vi "Core_Chem_User_Interface_v1.4.vi"() -> ()   [LabVIEW 2014] (continued)
    n188 = Decimal String To Number(string=w445) -> (number=w443:i32)  [unwired: 2 in, 1 out]
    n189 = call "Find_Data_SubVI.vi"("FGGA"=w553, "CO"=w552, "Ozone"=w551, "SO2"=w472) -> ("Output Value"=→"CPU Total %":dbl)  [unwired: 11 in]
    n190 = call "Find_Data_SubVI.vi"("FGGA"=w541, "CO"=w540, "Ozone"=w539, "SO2"=w538) -> ("Output Value"=→"MFM":dbl)  [unwired: 11 in]
    n191 = call "Find_Data_SubVI.vi"("FGGA"=w536, "CO"=w535, "Ozone"=w534, "SO2"=w533) -> ("Output Value"=w532:dbl)  [unwired: 11 in]
    n192 = call "Find_Data_SubVI.vi"("FGGA"=w521, "CO"=w524, "Ozone"=w519, "SO2"=w526) -> ("Output Value"=→"USB Disk Space Used %":dbl)  [unwired: 11 in]
    n193 = Not Equal To 0?(x=w532) -> (x != 0?=→"PTP Sync":bool)
    n194 = Add(x=w443, y=u32 2082844800) -> (x+y=w442:u32)
    n195 = Scan Value(string=w403, format string="%f") -> (value=→"MFC1 Cal Flow":dbl)  [unwired: 1 in, 1 out]
    n196 = Scan Value(string=w367, format string="%f") -> (value=w365:dbl)  [unwired: 1 in, 1 out]
    n197 = Scan Value(string=w366, format string="%f") -> (value=w363:dbl)  [unwired: 1 in, 1 out]
    n198 = Scan Value(string=w416, format string="%f") -> (value=→"Cell temperature":dbl)  [unwired: 1 in, 1 out]
    n199 = Scan Value(string=w417, format string="%f") -> (value=→"Cell pressure":dbl)  [unwired: 1 in, 1 out]
    n200 = Scan Value(string=w422, format string="%f") -> (value=→"CH4 Dry":dbl)  [unwired: 1 in, 1 out]
    n201 = Scan Value(string=w425, format string="%f") -> (value=→"CO2 Dry":dbl)  [unwired: 1 in, 1 out]
    n202 = Scan Value(string=w427, format string="%f") -> (value=→"H2O":dbl)  [unwired: 1 in, 1 out]
    n203 = Scan Value(string=w432, format string="%f") -> (value=→"CO2":dbl)  [unwired: 1 in, 1 out]
    n204 = Scan Value(string=w435, format string="%f") -> (value=→"CH4":dbl)  [unwired: 1 in, 1 out]
    n205 = Scan Value(string=w563, format string="%f") -> (value=→"Std\nContent (barG)":dbl)  [unwired: 1 in, 1 out]
    n206 = Scan Value(string=w523, format string="%d", default (0 dbl)=u32 0) -> (value=w577:u32)  [unwired: 1 out]
    n207 = Scan Value(string=w562, format string="%f") -> (value=→"N2\nContent (barG)":dbl)  [unwired: 1 in, 1 out]
    n208 = Scan Value(string=w564, format string="%f") -> (value=→"CO2\nContent (barG)":dbl)  [unwired: 1 in, 1 out]
    n209 = Scan Value(string=w570, format string="%f") -> (value=→"CO2 Pressure\nDelivery (PSIA)":dbl)  [unwired: 1 in, 1 out]
    n210 = To Time Stamp(1:w442) -> (0:w448:timestamp)
    n211 = Scan Value(string=w511, format string="%f") -> (value=→"Lamp Flow Controller":dbl)  [unwired: 1 in, 1 out]
    n212 = Scan Value(string=w380, format string="%f") -> (value=→"Raw Signal":dbl)  [unwired: 1 in, 1 out]
    n213 = Scan Value(string=w374, format string="%f") -> (value=→"Lamp Temperature":dbl)  [unwired: 1 in, 1 out]
    n214 = Scan Value(string=w399, format string="%f") -> (value=→"CO Concentration":dbl)  [unwired: 1 in, 1 out]
    n215 = Scan Value(string=w508, format string="%f") -> (value=→"Monochromator Flow":dbl)  [unwired: 1 in, 1 out]
    n216 = Scan Value(string=w507, format string="%f") -> (value=→"Fluorescence Cell Pressure":dbl)  [unwired: 1 in, 1 out]
    n217 = Not Equal To 0?(x=w577) -> (x != 0?=→"CO CAL Status":bool)
    n218 = call "ping.vi"("host"="192.168.101.17" ("Host IP Address")) -> ("found?"=w372:bool)  [unwired: 8 in, 2 out]
    n219 = Scan Value(string=w490, format string="%f") -> (value=→"TEI49C Sample Flow B":dbl)  [unwired: 1 in, 1 out]
    n220 = Scan Value(string=w492, format string="%f") -> (value=→"TEi49C Concentration":dbl)  [unwired: 1 in, 1 out]
    n221 = Scan Value(string=w491, format string="%f") -> (value=→"TEI49C Sample Flow A":dbl)  [unwired: 1 in, 1 out]
    n222 = Scan Value(string=w467, format string="%f") -> (value=w458:dbl)  [unwired: 1 in, 1 out]
    n223 = Scan Value(string=w466, format string="%f") -> (value=w451:dbl)  [unwired: 1 in, 1 out]
    n224 = Not Equal?(x=w457, y=w458) -> (x != y?=w463:bool)
    n225 = Not Equal?(x=w449, y=w451) -> (x != y?=w456:bool)
    n226 = case shown="True" w463 {
      tunnel: w464 -> [w638 w647]
      tunnel: w462 -> [w639 w646]
      tunnel: [w639 w645] -> w461
      tunnel: w448 -> [_ w641]
      tunnel: w458 -> [_ w642]
      tunnel: [w638 w644] -> w460
      tunnel: [w637 w643] -> w459
      tunnel: w458 -> [_ w643]
      tunnel: w457 -> [w637 _]
      frame False {
      }
      frame True {
        n227 = Bundle(w641, w642) -> (w640:cluster{timestamp, dbl})  [unwired: 1 in]
        n228 = Replace Array Subset(array=w647, new element=w640, index=w646) -> (w644:cluster{"time stamp":timestamp, "Y":dbl}[])
        n229 = Increment(x=w646) -> (x+1=w645:i32)
      }
    }
    "CO Sensitivity" <- w460
    n230 = case shown="True" w456 {
      tunnel: w455 -> [w627 w636]
      tunnel: w454 -> [w628 w635]
      tunnel: [w628 w634] -> w452
      tunnel: w448 -> [_ w633]
      tunnel: w451 -> [_ w632]
      tunnel: [w627 w631] -> w453
      tunnel: [w626 w630] -> w450
      tunnel: w451 -> [_ w630]
      tunnel: w449 -> [w626 _]
      frame False {
      }
      frame True {
        n231 = Bundle(w633, w632) -> (w629:cluster{timestamp, dbl})  [unwired: 1 in]
        n232 = Replace Array Subset(array=w636, new element=w629, index=w635) -> (w631:cluster{"time stamp":timestamp, "Y":dbl}[])
        n233 = Increment(x=w635) -> (x+1=w634:i32)
      }
    }
    "CO Zero" <- w453
    n234 = case shown="True" w372 {
      tunnel: w447 -> [_ w625]
      tunnel: [FALSE w622] -> w446
      frame False {
      }
      frame True {
        n235 = Select(t=FALSE, s=w625, f=TRUE) -> (s? t:f=w622:bool)
      }
    }
    "Network to cRIO live status" <- w446
    n236 = Bundle(w365, w363) -> (→"Ring Down Time RDA & RDB":cluster{dbl, dbl})  [unwired: 1 in]
    n237 = Wait (ms)(milliseconds to wait=u32 1000) -> ()  [unwired: 1 out]
  }
  n238 = while {
    stop <- FALSE stop-if-true
    # "Preflight Sub VI Descriptions"
    n239 = Wait (ms)(milliseconds to wait=u32 500) -> ()  [unwired: 1 out]
    n240 = case shown="True" "Line Lock Setting Change" {
      frame False {
      }
      frame True {
        n241 = call "FGGA Linelock Settings Procedures.vi"() -> ()  [unwired: 12 in]
      }
    }
  }
  n242 = while {
    stop <- FALSE stop-if-true
    # "Postflight Sub VI Descriptions"
    n243 = case shown="True" "Postflight Procedures" {
      frame False {
      }
      frame True {
        n244 = call "PostFlight Procedures.vi"() -> ()  [unwired: 12 in]
      }
    }
    n245 = Wait (ms)(milliseconds to wait=u32 500) -> ()  [unwired: 1 out]
  }
  n246 = while {
    stop <- FALSE stop-if-true
    # "Preflight Sub VI Descriptions"
    n247 = case shown="True" "Prepare Gases" {
      frame False {
      }
      frame True {
        n248 = call "CO Gas Preparation.vi"() -> ()  [unwired: 12 in]
      }
    }
    n249 = Wait (ms)(milliseconds to wait=u32 500) -> ()  [unwired: 1 out]
  }
  n250 = Obtain Queue(name (unnamed)="FGGA_Command", element data type=w55) -> (queue out=w2:refnum<queue>, error out=w1:errorcluster)  [unwired: 3 in, 1 out]
  n251 = while {
    shift-right: [w660] -> _
    shift-left: u8 1 -> [w661]
    tunnel: w2 -> [w658]
    tunnel: w1 -> [w657]
    stop <- FALSE stop-if-true
    # "FGGA pump synchronise to WoW Wait on Wheel Flag"
    n252 = Wait (ms)(milliseconds to wait=u32 1000) -> ()  [unwired: 1 out]
    n253 = case shown="True" "FGGA pump\nsync to WoW" {
      tunnel: [w664 w669] -> w660
      tunnel: w661 -> [w664 w668]
      tunnel: w658 -> [_ w667]
      tunnel: w657 -> [_ w666]
      frame False {
      }
      frame True {
        n254 = local read "WoW Flag"() -> (w665:string)
        n255 = Scan Value(string=w665, format string="%d", default (0 dbl)=u8 0) -> (value=w669:u8)  [unwired: 1 out]
        n256 = Not Equal?(x=w669, y=w668) -> (x != y?=w672:bool)
        n257 = case shown="True" w672 {
          tunnel: w669 -> [_ w675]
          tunnel: w667 -> [_ w674]
          tunnel: w666 -> [_ w673]
          frame False {
          }
          frame True {
            n258 = Equal?(x=w675, y=u8 0) -> (x = y?=w680:bool)
            n259 = case shown="True" w680 {
              selector: w680 -> [w682 w683]
              tunnel: [w682 w683] -> w676
              frame False {
              }
              frame True {
              }
            }
            n260 = local write "Manual FGGA Pump"(w676) -> ()
            n261 = Bundle(cluster=T4 {"Message"="", "Message Data"=variant} ("Message Cluster"), "Message"="FGGA_pump", "Message Data"=w676) -> (w677:T4)
            n262 = Enqueue Element(queue=w674, element=w677, error in (no error)=w673) -> ()  [unwired: 1 in, 3 out]
          }
        }
      }
    }
  }
  n263 = while {
    tunnel: w2 -> [w685]
    tunnel: w1 -> [w684]
    tunnel: [w687] -> _
    tunnel: w13 -> [w686]
    stop <- FALSE stop-if-true
    # "FGGA UI Event Handler Loop"
    n264 = event shown="[5] \"Confirm Flight Number\": Value Change" {
      selector: _ -> [_ _ _ _ _ _ _ _ _ _ _ _ _ _ _ _ _]
      dyn-events: _ -> [_ _ _ _ _ _ _ _ _ _ _ _ _ _ _ _ _]
      timeout: _ -> [_ _ _ _ _ _ _ _ _ _ _ _ _ _ _ _ _]
      tunnel: w685 -> [w695 w699 w706 w713 w720 w728 w742 w749 w768 w877 w1050 w1117 w1184 w1241 w1328 w1396 w1403]
      tunnel: w684 -> [w694 w698 w705 w712 w719 w727 w741 w748 w767 w876 w1049 w1116 w1183 w1240 w1327 w1395 w1402]
      tunnel: [w689 w697 w704 w711 w718 w726 w740 w747 w754 w840 w1042 w1109 w1176 w1227 w1314 w1394 w1401] -> w687
      tunnel: w686 -> [_ _ _ _ _ _ _ _ _ w864 _ _ _ _ _ _ _]
      event "eV1": Value Change {
        n265 = event-data() -> ("NewVal"=w692:bool)  [unwired: 1 in]
        n266 = Bundle(cluster=T4 {"Message"="", "Message Data"=variant} ("Message Cluster"), "Message"="V1", "Message Data"=w692) -> (w690:T4)
        n267 = Enqueue Element(queue=w695, element=w690, error in (no error)=w694) -> (error out=w689:errorcluster)  [unwired: 1 in, 2 out]
      }
      event "eV2": Value Change {
        n268 = event-data() -> ("NewVal"=w696:bool)  [unwired: 1 in]
        n269 = Bundle(cluster=T4 {"Message"="", "Message Data"=variant} ("Message Cluster"), "Message"="V2", "Message Data"=w696) -> (w700:T4)
        n270 = Enqueue Element(queue=w699, element=w700, error in (no error)=w698) -> (error out=w697:errorcluster)  [unwired: 1 in, 2 out]
      }
      event "eV3": Value Change {
        n271 = event-data() -> ("NewVal"=w703:bool)  [unwired: 1 in]
        n272 = Bundle(cluster=T4 {"Message"="", "Message Data"=variant} ("Message Cluster"), "Message"="V3", "Message Data"=w703) -> (w707:T4)
        n273 = Enqueue Element(queue=w706, element=w707, error in (no error)=w705) -> (error out=w704:errorcluster)  [unwired: 1 in, 2 out]
      }
      event "eV4": Value Change {
        n274 = event-data() -> ("NewVal"=w710:bool)  [unwired: 1 in]
        n275 = Bundle(cluster=T4 {"Message"="", "Message Data"=variant} ("Message Cluster"), "Message"="V4", "Message Data"=w710) -> (w714:T4)
        n276 = Enqueue Element(queue=w713, element=w714, error in (no error)=w712) -> (error out=w711:errorcluster)  [unwired: 1 in, 2 out]
      }
      event "Manual FGGA Pump": Value Change {
        n277 = event-data() -> ("NewVal"=w717:bool)  [unwired: 1 in]
        n278 = Bundle(cluster=T4 {"Message"="", "Message Data"=variant} ("Message Cluster"), "Message"="FGGA_pump", "Message Data"=w717) -> (w721:T4)
        n279 = Enqueue Element(queue=w720, element=w721, error in (no error)=w719) -> (error out=w718:errorcluster)  [unwired: 1 in, 2 out]
      }
      event "Confirm Flight Number": Value Change {
        n280 = event-data() -> ()  [unwired: 1 in, 6 out]
        n281 = flat-sequence {
          tunnel: w727 -> [w730]
          tunnel: w728 -> [w731]
          tunnel: [w731] -> w725
          tunnel: [w730] -> w724
          tunnel: [w733] -> w726
          tunnel: w725 -> [w735]
          tunnel: w724 -> [w734]
          frame #0 {
            n282 = local write "cRIO File IO Stop\n(USB Flash Drive Unmount)"(FALSE ("cRIO File IO Stop\n(USB Flash Drive Unmount)")) -> ()
          }
          frame #1 {
            n283 = local read "Flight Number"() -> (w732:string)
            n284 = Bundle(cluster=T4 {"Message"="", "Message Data"=variant} ("Message Cluster"), "Message"="Flight Number", "Message Data"=w732) -> (w736:T4)
            n285 = Enqueue Element(queue=w735, element=w736, error in (no error)=w734) -> (error out=w733:errorcluster)  [unwired: 1 in, 2 out]
          }
        }
      }
      event "FGGA Restart": Value Change {
        n286 = event-data() -> ("NewVal"=w739:bool)  [unwired: 1 in]
        n287 = Bundle(cluster=T4 {"Message"="", "Message Data"=variant} ("Message Cluster"), "Message"="FGGA_restart", "Message Data"=w739) -> (w743:T4)
        n288 = Enqueue Element(queue=w742, element=w743, error in (no error)=w741) -> (error out=w740:errorcluster)  [unwired: 1 in, 2 out]
      }
      event "cRIO File IO Stop\n(USB Flash Drive Unmount)": Value Change {
        n289 = event-data() -> ("NewVal"=w746:bool)  [unwired: 1 in]
        n290 = Bundle(cluster=T4 {"Message"="", "Message Data"=variant} ("Message Cluster"), "Message"="Stop File Write", "Message Data"=w746) -> (w750:T4)
        n291 = Enqueue Element(queue=w749, element=w750, error in (no error)=w748) -> (error out=w747:errorcluster)  [unwired: 1 in, 2 out]
      }
      event "High Cal": Value Change {
        n292 = event-data() -> ()  [unwired: 1 in, 1 out]
        n293 = flat-sequence {
          tunnel: w768 -> [w773]
          tunnel: w767 -> [w772]
          tunnel: [w771] -> w766
          tunnel: [w770] -> w765
          tunnel: w766 -> [w789]
          tunnel: w765 -> [w788]
          tunnel: [w786] -> w763
          tunnel: [w785] -> w761
          tunnel: [w794] -> w764
          tunnel: w763 -> [w794]
          tunnel: [w793] -> w762
          tunnel: w761 -> [w793]
          tunnel: w764 -> [w804]
          tunnel: w762 -> [w803]
          tunnel: [w801] -> w759
          tunnel: [w800] -> w757
          tunnel: [w810] -> w760
          tunnel: w759 -> [w810]
          tunnel: [w809] -> w758
          tunnel: w757 -> [w809]
          tunnel: w760 -> [w820]
          tunnel: w758 -> [w819]
          tunnel: [w817] -> w756
          tunnel: [w816] -> w755
          tunnel: w756 -> [w834]
          tunnel: w755 -> [w833]
          tunnel: [w831] -> w753
          tunnel: [w839] -> w754
          tunnel: w753 -> [w839]
          frame #0 {
            w769 = TRUE
            n294 = Cluster To Array(cluster=T11 {"Message"="V2", "Message 2"="V3", "Message 3"="V4"}) -> (array=w774:string[])
            n295 = for {
              tunnel: w774 -> [w781] mode=indexing
              tunnel: w773 -> [w780]
              tunnel: w772 -> [w779]
              tunnel: [w778] -> w771
              tunnel: [w777] -> w770
              tunnel: w769 -> [w776]
              n296 = Bundle(cluster=T4 {"Message"="", "Message Data"=variant} ("Message Cluster"), "Message"=w781, "Message Data"=w776) -> (w783:T4)
              n297 = Enqueue Element(queue=w780, element=w783, error in (no error)=w779) -> (queue out=w778:refnum<queue>, error out=w777:errorcluster)  [unwired: 1 in, 1 out]
            }
            n298 = local write "eV2"(w769) -> ()
            n299 = local write "eV4"(w769) -> ()
            n300 = local write "eV3"(w769) -> ()
          }
          frame #1 {
            n301 = local read "MFC_1 User Set Value"() -> (w784:dbl)
            n302 = local write "MFC_1\nSLPM Value"(w784) -> ()
            n303 = Bundle(cluster=T4 {"Message"="", "Message Data"=variant} ("Message Cluster"), "Message"="MFC_1", "Message Data"=w784) -> (w787:T4)
            n304 = Enqueue Element(queue=w789, element=w787, error in (no error)=w788) -> (queue out=w786:refnum<queue>, error out=w785:errorcluster)  [unwired: 1 in, 1 out]
          }
          frame #2 {
            n305 = for {
              N: 45 -> [w798]
              i -> [w797]
              n306 = Subtract(x=w798, y=w797) -> (x-y=w796:i32)
              n307 = Decrement(x=w796) -> (x-1=→"High Cal\nFlush Time Remain (sec)":i32)
              n308 = Wait (ms)(milliseconds to wait=u32 1000) -> ()  [unwired: 1 out]
            }
          }
          frame #3 {
            w802 = TRUE
            n309 = Bundle(cluster=T4 {"Message"="", "Message Data"=variant} ("Message Cluster"), "Message"="V1", "Message Data"=w802) -> (w805:T4)
            n310 = local write "eV1"(w802) -> ()
            n311 = Enqueue Element(queue=w804, element=w805, error in (no error)=w803) -> (queue out=w801:refnum<queue>, error out=w800:errorcluster)  [unwired: 1 in, 1 out]
          }
          frame #4 {
            n312 = for {
              N: 60 -> [w814]
              i -> [w813]
              n313 = Subtract(x=w814, y=w813) -> (x-y=w812:i32)
              n314 = Decrement(x=w812) -> (x-1=→"High Cal\nCal Time Remain (sec)":i32)
              n315 = Wait (ms)(milliseconds to wait=u32 1000) -> ()  [unwired: 1 out]
            }
          }
          frame #5 {
            w818 = FALSE
            n316 = Cluster To Array(cluster=T12 {"Message"="V2", "Message 2"="V3", "Message 3"="V4", "Message 4"="V1"}) -> (array=w821:string[])
            n317 = for {
              tunnel: w821 -> [w828] mode=indexing
              tunnel: [w827] -> w817
              tunnel: [w826] -> w816
              tunnel: w818 -> [w825]
              tunnel: w820 -> [w824]
              tunnel: w819 -> [w823]
              n318 = Bundle(cluster=T4 {"Message"="", "Message Data"=variant} ("Message Cluster"), "Message"=w828, "Message Data"=w825) -> (w830:T4)
              n319 = Enqueue Element(queue=w824, element=w830, error in (no error)=w823) -> (queue out=w827:refnum<queue>, error out=w826:errorcluster)  [unwired: 1 in, 1 out]
            }
            n320 = local write "eV2"(w818) -> ()
            n321 = local write "eV4"(w818) -> ()
            n322 = local write "eV3"(w818) -> ()
            n323 = local write "eV1"(w818) -> ()
          }
          frame #6 {
            w832 = 0.0 ("MFC_1\nSLPM Value")
            n324 = local write "MFC_1\nSLPM Value"(w832) -> ()
            n325 = Bundle(cluster=T4 {"Message"="", "Message Data"=variant} ("Message Cluster"), "Message"="MFC_1", "Message Data"=w832) -> (w836:T4)
            n326 = Enqueue Element(queue=w834, element=w836, error in (no error)=w833) -> (error out=w831:errorcluster)  [unwired: 1 in, 2 out]
          }
          frame #7 {
            n327 = local write "High Cal"(FALSE ("High Cal")) -> ()
          }
        }
      }
      event "Span Cal - \nHigh Cal, CO Cal, Low Cal": Value Change {
        n328 = event-data() -> ()  [unwired: 1 in, 1 out]
        n329 = flat-sequence {
          tunnel: w877 -> [w883]
          tunnel: w876 -> [w882]
          tunnel: [w881] -> w875
          tunnel: [w880] -> w874
          tunnel: w875 -> [w899]
          tunnel: w874 -> [w898]
          tunnel: [w896] -> w872
          tunnel: [w895] -> w870
          tunnel: [w904] -> w873
          tunnel: w872 -> [w904]
          tunnel: [w903] -> w871
          tunnel: w870 -> [w903]
          tunnel: w873 -> [w910]
          tunnel: w871 -> [w911]
          tunnel: [w911] -> w846
          tunnel: w864 -> [w912]
          tunnel: [w912] -> w844
          tunnel: [w910] -> w842
          tunnel: w846 -> [w920]
          tunnel: [w920] -> w845
          tunnel: w844 -> [w919]
          tunnel: [w919] -> w843
          tunnel: w842 -> [w917]
          tunnel: [w917] -> w841
          tunnel: [w921] -> w863
          tunnel: w845 -> [w924]
          tunnel: [w923] -> w862
          tunnel: w843 -> [w933]
          tunnel: w841 -> [w922]
          tunnel: [w936] -> w869
          tunnel: w863 -> [w936]
          tunnel: [w935] -> w868
          tunnel: w862 -> [w935]
          tunnel: w869 -> [w946]
          tunnel: w868 -> [w945]
          tunnel: [w943] -> w867
          tunnel: [w942] -> w866
          tunnel: w867 -> [w961]
          tunnel: w866 -> [w960]
          tunnel: [w958] -> w865
          tunnel: [w957] -> w859
          tunnel: w865 -> [w967]
          tunnel: [w967] -> w861
          tunnel: [w965] -> w860
          tunnel: w859 -> [w965]
          tunnel: w861 -> [w972]
          tunnel: w860 -> [w974]
          tunnel: [w971] -> w858
          tunnel: [w968] -> w857
          tunnel: w858 -> [w988]
          tunnel: w857 -> [w986]
          tunnel: [w985] -> w856
          tunnel: [w984] -> w853
          tunnel: w856 -> [w993]
          tunnel: [w993] -> w855
          tunnel: [w992] -> w854
          tunnel: w853 -> [w992]
          tunnel: w855 -> [w1005]
          tunnel: w854 -> [w1003]
          tunnel: [w1001] -> w851
          tunnel: [w1000] -> w849
          tunnel: [w1009] -> w852
          tunnel: w851 -> [w1009]
          tunnel: [w1008] -> w850
          tunnel: w849 -> [w1008]
          tunnel: w852 -> [w1020]
          tunnel: w850 -> [w1019]
          tunnel: [w1017] -> w848
          tunnel: [w1016] -> w847
          tunnel: w848 -> [w1035]
          tunnel: w847 -> [w1034]
          tunnel: [w1031] -> w840
          frame #0 {
            w879 = TRUE
            n330 = Cluster To Array(cluster=T11 {"Message"="V2", "Message 2"="V3", "Message 3"="V4"}) -> (array=w884:string[])
            n331 = for {
              tunnel: w884 -> [w891] mode=indexing
              tunnel: w883 -> [w890]
              tunnel: w882 -> [w889]
              tunnel: [w888] -> w881
              tunnel: [w887] -> w880
              tunnel: w879 -> [w886]
              n332 = Bundle(cluster=T4 {"Message"="", "Message Data"=variant} ("Message Cluster"), "Message"=w891, "Message Data"=w886) -> (w893:T4)
              n333 = Enqueue Element(queue=w890, element=w893, error in (no error)=w889) -> (queue out=w888:refnum<queue>, error out=w887:errorcluster)  [unwired: 1 in, 1 out]
            }
            n334 = local write "High Cal"(TRUE ("High Cal")) -> ()
            n335 = local write "eV2"(w879) -> ()
            n336 = local write "eV4"(w879) -> ()
            n337 = local write "eV3"(w879) -> ()
          }
          frame #1 {
            n338 = local read "MFC_1 User Set Value"() -> (w894:dbl)
            n339 = local write "MFC_1\nSLPM Value"(w894) -> ()
            n340 = Bundle(cluster=T4 {"Message"="", "Message Data"=variant} ("Message Cluster"), "Message"="MFC_1", "Message Data"=w894) -> (w897:T4)
            n341 = Enqueue Element(queue=w899, element=w897, error in (no error)=w898) -> (queue out=w896:refnum<queue>, error out=w895:errorcluster)  [unwired: 1 in, 1 out]
          }
          frame #2 {
            n342 = for {
              N: 45 -> [w908]
              i -> [w907]
              n343 = Subtract(x=w908, y=w907) -> (x-y=w906:i32)
              n344 = Decrement(x=w906) -> (x-1=w905:i32)
              n345 = local write "High Cal\nFlush Time Remain (sec)"(w905) -> ()
              n346 = Wait (ms)(milliseconds to wait=u32 1000) -> ()  [unwired: 1 out]
            }
          }
          frame #3 {
            n347 = Bundle(cluster=T4 {"Message"="", "Message Data"=variant} ("Message Cluster"), "Message"="CO CAL", "Message Data"=TRUE) -> (w914:T4)
            n348 = Enqueue Element(queue=w912, element=w914) -> ()  [unwired: 2 in, 3 out]
          }
          frame #4 {
            # "To Ensure\nCO CAL\nis certain"
            n349 = Wait (ms)(milliseconds to wait=u32 1000) -> ()  [unwired: 1 out]
          }
          frame #5 {
            w928 = TRUE
            n350 = Bundle(cluster=T4 {"Message"="", "Message Data"=variant} ("Message Cluster"), "Message"="CO CAL", "Message Data"=FALSE) -> (w929:T4)
            n351 = Bundle(cluster=T4 {"Message"="", "Message Data"=variant} ("Message Cluster"), "Message"="V1", "Message Data"=w928) -> (w927:T4)
            n352 = local write "eV1"(w928) -> ()
            n353 = Enqueue Element(queue=w933, element=w929) -> ()  [unwired: 2 in, 3 out]
            n354 = Enqueue Element(queue=w922, element=w927, error in (no error)=w924) -> (queue out=w921:refnum<queue>, error out=w923:errorcluster)  [unwired: 1 in, 1 out]
          }
          frame #6 {
            n355 = for {
              N: 60 -> [w940]
              i -> [w939]
              n356 = Subtract(x=w940, y=w939) -> (x-y=w938:i32)
              n357 = Decrement(x=w938) -> (x-1=w937:i32)
              n358 = local write "High Cal\nCal Time Remain (sec)"(w937) -> ()
              n359 = Wait (ms)(milliseconds to wait=u32 1000) -> ()  [unwired: 1 out]
            }
          }
          frame #7 {
            w944 = FALSE
            n360 = Cluster To Array(cluster=T12 {"Message"="V2", "Message 2"="V3", "Message 3"="V4", "Message 4"="V1"}) -> (array=w947:string[])
            n361 = for {
              tunnel: w947 -> [w954] mode=indexing
              tunnel: [w953] -> w943
              tunnel: [w952] -> w942
              tunnel: w944 -> [w951]
              tunnel: w946 -> [w950]
              tunnel: w945 -> [w949]
              n362 = Bundle(cluster=T4 {"Message"="", "Message Data"=variant} ("Message Cluster"), "Message"=w954, "Message Data"=w951) -> (w956:T4)
              n363 = Enqueue Element(queue=w950, element=w956, error in (no error)=w949) -> (queue out=w953:refnum<queue>, error out=w952:errorcluster)  [unwired: 1 in, 1 out]
            }
            n364 = local write "eV2"(w944) -> ()
            n365 = local write "eV4"(w944) -> ()
            n366 = local write "eV3"(w944) -> ()
            n367 = local write "eV1"(w944) -> ()
          }
          frame #8 {
            w959 = 0.0 ("MFC_1\nSLPM Value")
            n368 = local write "MFC_1\nSLPM Value"(w959) -> ()
            n369 = Bundle(cluster=T4 {"Message"="", "Message Data"=variant} ("Message Cluster"), "Message"="MFC_1", "Message Data"=w959) -> (w963:T4)
            n370 = Enqueue Element(queue=w961, element=w963, error in (no error)=w960) -> (queue out=w957:refnum<queue>, error out=w958:errorcluster)  [unwired: 1 in, 1 out]
          }
          frame #9 {
            n371 = local write "High Cal"(FALSE ("High Cal")) -> ()
          }
          frame #10 {
            w969 = TRUE
            n372 = Cluster To Array(cluster=cluster{"Message":string, "Message 3":string} {"Message"="V2", "Message 3"="V4"}) -> (array=w975:string[])
            n373 = for {
              tunnel: w975 -> [w981] mode=indexing
              tunnel: w974 -> [w980]
              tunnel: [w979] -> w968
              tunnel: [w978] -> w971
              tunnel: w969 -> [w977]
              tunnel: w972 -> [w976]
              n374 = Bundle(cluster=T4 {"Message"="", "Message Data"=variant} ("Message Cluster"), "Message"=w981, "Message Data"=w977) -> (w983:T4)
              n375 = Enqueue Element(queue=w980, element=w983, error in (no error)=w976) -> (queue out=w979:refnum<queue>, error out=w978:errorcluster)  [unwired: 1 in, 1 out]
            }
            n376 = local write "eV4"(w969) -> ()
            n377 = local write "eV2"(w969) -> ()
            n378 = local write "Low Cal"(TRUE ("Low Cal")) -> ()
          }
          frame #11 {
            n379 = local read "MFC_1 User Set Value"() -> (w989:dbl)
            n380 = local write "MFC_1\nSLPM Value"(w989) -> ()
            n381 = Bundle(cluster=T4 {"Message"="", "Message Data"=variant} ("Message Cluster"), "Message"="MFC_1", "Message Data"=w989) -> (w990:T4)
            n382 = Enqueue Element(queue=w986, element=w990, error in (no error)=w988) -> (queue out=w985:refnum<queue>, error out=w984:errorcluster)  [unwired: 1 in, 1 out]
          }
          frame #12 {
            n383 = for {
              N: 45 -> [w998]
              i -> [w997]
              n384 = Subtract(x=w998, y=w997) -> (x-y=w996:i32)
              n385 = Decrement(x=w996) -> (x-1=w995:i32)
              n386 = local write "Low Cal\nFlush Time Remain (sec)"(w995) -> ()
              n387 = Wait (ms)(milliseconds to wait=u32 1000) -> ()  [unwired: 1 out]
            }
          }
          frame #13 {
            w1002 = TRUE
            n388 = local write "eV1"(w1002) -> ()
            n389 = Bundle(cluster=T4 {"Message"="", "Message Data"=variant} ("Message Cluster"), "Message"="V1", "Message Data"=w1002) -> (w1006:T4)
            n390 = Enqueue Element(queue=w1005, element=w1006, error in (no error)=w1003) -> (queue out=w1001:refnum<queue>, error out=w1000:errorcluster)  [unwired: 1 in, 1 out]
          }
          frame #14 {
            n391 = for {
              N: 60 -> [w1014]
              i -> [w1013]
              n392 = Subtract(x=w1014, y=w1013) -> (x-y=w1012:i32)
              n393 = Decrement(x=w1012) -> (x-1=w1011:i32)
              n394 = local write "Low Cal\nCal Time Remain (sec)"(w1011) -> ()
              n395 = Wait (ms)(milliseconds to wait=u32 1000) -> ()  [unwired: 1 out]
            }
          }
          frame #15 {
            w1018 = FALSE
            n396 = Cluster To Array(cluster=T13 {"Message"="V2", "Message 3"="V4", "Message 4"="V1"}) -> (array=w1021:string[])
            n397 = local write "eV1"(w1018) -> ()
            n398 = local write "eV2"(w1018) -> ()
            n399 = local write "eV4"(w1018) -> ()
            n400 = for {
              tunnel: w1021 -> [w1028] mode=indexing
              tunnel: [w1027] -> w1017
              tunnel: [w1026] -> w1016
              tunnel: w1018 -> [w1025]
              tunnel: w1020 -> [w1024]
              tunnel: w1019 -> [w1023]
              n401 = Bundle(cluster=T4 {"Message"="", "Message Data"=variant} ("Message Cluster"), "Message"=w1028, "Message Data"=w1025) -> (w1030:T4)
              n402 = Enqueue Element(queue=w1024, element=w1030, error in (no error)=w1023) -> (queue out=w1027:refnum<queue>, error out=w1026:errorcluster)  [unwired: 1 in, 1 out]
            }
          }
          frame #16 {
            w1032 = FALSE
            w1033 = 0.0 ("MFC_1\nSLPM Value")
            n403 = local write "Span Cal - \nHigh Cal, CO Cal, Low Cal"(w1032) -> ()
            n404 = local write "MFC_1\nSLPM Value"(w1033) -> ()
            n405 = local write "Low Cal"(w1032) -> ()
            n406 = Bundle(cluster=T4 {"Message"="", "Message Data"=variant} ("Message Cluster"), "Message"="MFC_1", "Message Data"=w1033) -> (w1037:T4)
            n407 = Enqueue Element(queue=w1035, element=w1037, error in (no error)=w1034) -> (error out=w1031:errorcluster)  [unwired: 1 in, 2 out]
          }
        }
      }
      event "Flush High Tank": Value Change {
        n408 = event-data() -> ()  [unwired: 1 in, 1 out]
        n409 = flat-sequence {
          tunnel: w1050 -> [w1055]
          tunnel: w1049 -> [w1054]
          tunnel: [w1053] -> w1048
          tunnel: [w1052] -> w1047
          tunnel: w1048 -> [w1071]
          tunnel: w1047 -> [w1070]
          tunnel: [w1068] -> w1046
          tunnel: [w1067] -> w1045
          tunnel: w1046 -> [w1074]
          tunnel: w1045 -> [w1075]
          tunnel: [w1075] -> w1040
          tunnel: [w1074] -> w1039
          tunnel: [w1085] -> w1044
          tunnel: [w1084] -> w1043
          tunnel: w1040 -> [w1083]
          tunnel: w1039 -> [w1082]
          tunnel: w1044 -> [w1100]
          tunnel: w1043 -> [w1099]
          tunnel: [w1097] -> w1041
          tunnel: [w1105] -> w1042
          tunnel: w1041 -> [w1105]
          frame #0 {
            w1051 = TRUE
            n410 = Cluster To Array(cluster=T11 {"Message"="V2", "Message 2"="V3", "Message 3"="V4"}) -> (array=w1056:string[])
            n411 = for {
              tunnel: w1056 -> [w1063] mode=indexing
              tunnel: w1055 -> [w1062]
              tunnel: w1054 -> [w1061]
              tunnel: [w1060] -> w1053
              tunnel: [w1059] -> w1052
              tunnel: w1051 -> [w1058]
              n412 = Bundle(cluster=T4 {"Message"="", "Message Data"=variant} ("Message Cluster"), "Message"=w1063, "Message Data"=w1058) -> (w1065:T4)
              n413 = Enqueue Element(queue=w1062, element=w1065, error in (no error)=w1061) -> (queue out=w1060:refnum<queue>, error out=w1059:errorcluster)  [unwired: 1 in, 1 out]
            }
            n414 = local write "eV2"(w1051) -> ()
            n415 = local write "eV4"(w1051) -> ()
            n416 = local write "eV3"(w1051) -> ()
          }
          frame #1 {
            n417 = local read "MFC_1 User Set Value"() -> (w1066:dbl)
            n418 = local write "MFC_1\nSLPM Value"(w1066) -> ()
            n419 = Bundle(cluster=T4 {"Message"="", "Message Data"=variant} ("Message Cluster"), "Message"="MFC_1", "Message Data"=w1066) -> (w1069:T4)
            n420 = Enqueue Element(queue=w1071, element=w1069, error in (no error)=w1070) -> (queue out=w1068:refnum<queue>, error out=w1067:errorcluster)  [unwired: 1 in, 1 out]
          }
          frame #2 {
            n421 = for {
              N: 15 -> [w1080]
              i -> [w1079]
              n422 = Subtract(x=w1080, y=w1079) -> (x-y=w1078:i32)
              n423 = Decrement(x=w1078) -> (x-1=→"Flush High Tank\nTime Remain (sec)":i32)
              n424 = Wait (ms)(milliseconds to wait=u32 1000) -> ()  [unwired: 1 out]
            }
          }
          frame #3 {
            w1086 = FALSE
            n425 = Cluster To Array(cluster=T11 {"Message"="V2", "Message 2"="V3", "Message 3"="V4"}) -> (array=w1087:string[])
            n426 = for {
              tunnel: w1087 -> [w1094] mode=indexing
              tunnel: [w1093] -> w1085
              tunnel: [w1092] -> w1084
              tunnel: w1086 -> [w1091]
              tunnel: w1082 -> [w1090]
              tunnel: w1083 -> [w1089]
              n427 = Bundle(cluster=T4 {"Message"="", "Message Data"=variant} ("Message Cluster"), "Message"=w1094, "Message Data"=w1091) -> (w1096:T4)
              n428 = Enqueue Element(queue=w1090, element=w1096, error in (no error)=w1089) -> (queue out=w1093:refnum<queue>, error out=w1092:errorcluster)  [unwired: 1 in, 1 out]
            }
            n429 = local write "eV2"(w1086) -> ()
            n430 = local write "eV4"(w1086) -> ()
            n431 = local write "eV3"(w1086) -> ()
          }
          frame #4 {
            w1098 = 0.0 ("MFC_1\nSLPM Value")
            n432 = local write "MFC_1\nSLPM Value"(w1098) -> ()
            n433 = Bundle(cluster=T4 {"Message"="", "Message Data"=variant} ("Message Cluster"), "Message"="MFC_1", "Message Data"=w1098) -> (w1102:T4)
            n434 = Enqueue Element(queue=w1100, element=w1102, error in (no error)=w1099) -> (error out=w1097:errorcluster)  [unwired: 1 in, 2 out]
          }
          frame #5 {
            n435 = local write "Flush High Tank"(FALSE ("High Cal")) -> ()
          }
        }
      }
      event "Flush Low Tank": Value Change {
        n436 = event-data() -> ()  [unwired: 1 in, 1 out]
        n437 = flat-sequence {
          tunnel: w1117 -> [w1122]
          tunnel: w1116 -> [w1121]
          tunnel: [w1120] -> w1115
          tunnel: [w1119] -> w1114
          tunnel: w1115 -> [w1138]
          tunnel: w1114 -> [w1137]
          tunnel: [w1135] -> w1113
          tunnel: [w1134] -> w1112
          tunnel: w1113 -> [w1141]
          tunnel: w1112 -> [w1142]
          tunnel: [w1142] -> w1107
          tunnel: [w1141] -> w1106
          tunnel: [w1152] -> w1111
          tunnel: [w1151] -> w1110
          tunnel: w1107 -> [w1150]
          tunnel: w1106 -> [w1149]
          tunnel: w1111 -> [w1167]
          tunnel: w1110 -> [w1166]
          tunnel: [w1164] -> w1108
          tunnel: [w1172] -> w1109
          tunnel: w1108 -> [w1172]
          frame #0 {
            w1118 = TRUE
            n438 = Cluster To Array(cluster=cluster{"Message":string, "Message 3":string} {"Message"="V2", "Message 3"="V4"}) -> (array=w1123:string[])
            n439 = for {
              tunnel: w1123 -> [w1130] mode=indexing
              tunnel: w1122 -> [w1129]
              tunnel: w1121 -> [w1128]
              tunnel: [w1127] -> w1120
              tunnel: [w1126] -> w1119
              tunnel: w1118 -> [w1125]
              n440 = Bundle(cluster=T4 {"Message"="", "Message Data"=variant} ("Message Cluster"), "Message"=w1130, "Message Data"=w1125) -> (w1132:T4)
              n441 = Enqueue Element(queue=w1129, element=w1132, error in (no error)=w1128) -> (queue out=w1127:refnum<queue>, error out=w1126:errorcluster)  [unwired: 1 in, 1 out]
            }
            n442 = local write "eV2"(w1118) -> ()
            n443 = local write "eV4"(w1118) -> ()
          }
          frame #1 {
            n444 = local read "MFC_1 User Set Value"() -> (w1133:dbl)
            n445 = local write "MFC_1\nSLPM Value"(w1133) -> ()
            n446 = Bundle(cluster=T4 {"Message"="", "Message Data"=variant} ("Message Cluster"), "Message"="MFC_1", "Message Data"=w1133) -> (w1136:T4)
            n447 = Enqueue Element(queue=w1138, element=w1136, error in (no error)=w1137) -> (queue out=w1135:refnum<queue>, error out=w1134:errorcluster)  [unwired: 1 in, 1 out]
          }
          frame #2 {
            n448 = for {
              N: 15 -> [w1147]
              i -> [w1146]
              n449 = Subtract(x=w1147, y=w1146) -> (x-y=w1145:i32)
              n450 = Decrement(x=w1145) -> (x-1=→"Flush Low Tank\nTime Remain (sec)":i32)
              n451 = Wait (ms)(milliseconds to wait=u32 1000) -> ()  [unwired: 1 out]
            }
          }
          frame #3 {
            w1153 = FALSE
            n452 = Cluster To Array(cluster=cluster{"Message":string, "Message 3":string} {"Message"="V2", "Message 3"="V4"}) -> (array=w1154:string[])
            n453 = for {
              tunnel: w1154 -> [w1161] mode=indexing
              tunnel: [w1160] -> w1152
              tunnel: [w1159] -> w1151
              tunnel: w1153 -> [w1158]
              tunnel: w1149 -> [w1157]
              tunnel: w1150 -> [w1156]
              n454 = Bundle(cluster=T4 {"Message"="", "Message Data"=variant} ("Message Cluster"), "Message"=w1161, "Message Data"=w1158) -> (w1163:T4)
              n455 = Enqueue Element(queue=w1157, element=w1163, error in (no error)=w1156) -> (queue out=w1160:refnum<queue>, error out=w1159:errorcluster)  [unwired: 1 in, 1 out]
            }
            n456 = local write "eV2"(w1153) -> ()
            n457 = local write "eV4"(w1153) -> ()
          }
          frame #4 {
            w1165 = 0.0 ("MFC_1\nSLPM Value")
            n458 = local write "MFC_1\nSLPM Value"(w1165) -> ()
            n459 = Bundle(cluster=T4 {"Message"="", "Message Data"=variant} ("Message Cluster"), "Message"="MFC_1", "Message Data"=w1165) -> (w1169:T4)
            n460 = Enqueue Element(queue=w1167, element=w1169, error in (no error)=w1166) -> (error out=w1164:errorcluster)  [unwired: 1 in, 2 out]
          }
          frame #5 {
            n461 = local write "Flush Low Tank"(FALSE ("High Cal")) -> ()
          }
        }
      }
      event "Flush Target Tank": Value Change {
        n462 = event-data() -> ()  [unwired: 1 in, 1 out]
        n463 = flat-sequence {
          tunnel: w1184 -> [w1192]
          tunnel: w1183 -> [w1191]
          tunnel: [w1190] -> w1182
          tunnel: [w1189] -> w1181
          tunnel: w1182 -> [w1198]
          tunnel: w1181 -> [w1197]
          tunnel: [w1195] -> w1180
          tunnel: [w1194] -> w1179
          tunnel: w1180 -> [w1201]
          tunnel: w1179 -> [w1202]
          tunnel: [w1202] -> w1174
          tunnel: [w1201] -> w1173
          tunnel: [w1215] -> w1178
          tunnel: [w1214] -> w1177
          tunnel: w1174 -> [w1213]
          tunnel: w1173 -> [w1212]
          tunnel: w1178 -> [w1220]
          tunnel: w1177 -> [w1219]
          tunnel: [w1217] -> w1175
          tunnel: [w1225] -> w1176
          tunnel: w1175 -> [w1225]
          frame #0 {
            w1188 = TRUE
            n464 = local write "eV4"(w1188) -> ()
            n465 = Bundle(cluster=T4 {"Message"="", "Message Data"=variant} ("Message Cluster"), "Message"="V4" ("Message 3"), "Message Data"=w1188) -> (w1187:T4)
            n466 = Enqueue Element(queue=w1192, element=w1187, error in (no error)=w1191) -> (queue out=w1190:refnum<queue>, error out=w1189:errorcluster)  [unwired: 1 in, 1 out]
          }
          frame #1 {
            n467 = local read "MFC_1 User Set Value"() -> (w1193:dbl)
            n468 = local write "MFC_1\nSLPM Value"(w1193) -> ()
            n469 = Bundle(cluster=T4 {"Message"="", "Message Data"=variant} ("Message Cluster"), "Message"="MFC_1", "Message Data"=w1193) -> (w1196:T4)
            n470 = Enqueue Element(queue=w1198, element=w1196, error in (no error)=w1197) -> (queue out=w1195:refnum<queue>, error out=w1194:errorcluster)  [unwired: 1 in, 1 out]
          }
          frame #2 {
            n471 = for {
              N: 15 -> [w1207]
              i -> [w1206]
              n472 = Subtract(x=w1207, y=w1206) -> (x-y=w1205:i32)
              n473 = Decrement(x=w1205) -> (x-1=→"Flush Target Tank\nTime Remain (sec)":i32)
              n474 = Wait (ms)(milliseconds to wait=u32 1000) -> ()  [unwired: 1 out]
            }
          }
          frame #3 {
            w1216 = FALSE
            n475 = Bundle(cluster=T4 {"Message"="", "Message Data"=variant} ("Message Cluster"), "Message"="V4" ("Message 3"), "Message Data"=w1216) -> (w1211:T4)
            n476 = local write "eV4"(w1216) -> ()
            n477 = Enqueue Element(queue=w1212, element=w1211, error in (no error)=w1213) -> (queue out=w1215:refnum<queue>, error out=w1214:errorcluster)  [unwired: 1 in, 1 out]
          }
          frame #4 {
            w1218 = 0.0 ("MFC_1\nSLPM Value")
            n478 = local write "MFC_1\nSLPM Value"(w1218) -> ()
            n479 = Bundle(cluster=T4 {"Message"="", "Message Data"=variant} ("Message Cluster"), "Message"="MFC_1", "Message Data"=w1218) -> (w1222:T4)
            n480 = Enqueue Element(queue=w1220, element=w1222, error in (no error)=w1219) -> (error out=w1217:errorcluster)  [unwired: 1 in, 2 out]
          }
          frame #5 {
            n481 = local write "Flush Target Tank"(FALSE ("High Cal")) -> ()
          }
        }
      }
      event "Low Cal": Value Change {
        n482 = event-data() -> ()  [unwired: 1 in, 1 out]
        n483 = flat-sequence {
          tunnel: w1241 -> [w1246]
          tunnel: w1240 -> [w1245]
          tunnel: [w1244] -> w1239
          tunnel: [w1243] -> w1238
          tunnel: w1239 -> [w1262]
          tunnel: w1238 -> [w1261]
          tunnel: [w1259] -> w1236
          tunnel: [w1258] -> w1234
          tunnel: [w1267] -> w1237
          tunnel: w1236 -> [w1267]
          tunnel: [w1266] -> w1235
          tunnel: w1234 -> [w1266]
          tunnel: w1237 -> [w1277]
          tunnel: w1235 -> [w1276]
          tunnel: [w1274] -> w1232
          tunnel: [w1273] -> w1230
          tunnel: [w1283] -> w1233
          tunnel: w1232 -> [w1283]
          tunnel: [w1282] -> w1231
          tunnel: w1230 -> [w1282]
          tunnel: w1233 -> [w1293]
          tunnel: w1231 -> [w1292]
          tunnel: [w1290] -> w1229
          tunnel: [w1289] -> w1228
          tunnel: w1229 -> [w1307]
          tunnel: w1228 -> [w1306]
          tunnel: [w1304] -> w1226
          tunnel: [w1312] -> w1227
          tunnel: w1226 -> [w1312]
          frame #0 {
            w1242 = TRUE
            n484 = Cluster To Array(cluster=cluster{"Message":string, "Message 3":string} {"Message"="V2", "Message 3"="V4"}) -> (array=w1247:string[])
            n485 = for {
              tunnel: w1247 -> [w1254] mode=indexing
              tunnel: w1246 -> [w1253]
              tunnel: w1245 -> [w1252]
              tunnel: [w1251] -> w1244
              tunnel: [w1250] -> w1243
              tunnel: w1242 -> [w1249]
              n486 = Bundle(cluster=T4 {"Message"="", "Message Data"=variant} ("Message Cluster"), "Message"=w1254, "Message Data"=w1249) -> (w1256:T4)
              n487 = Enqueue Element(queue=w1253, element=w1256, error in (no error)=w1252) -> (queue out=w1251:refnum<queue>, error out=w1250:errorcluster)  [unwired: 1 in, 1 out]
            }
            n488 = local write "eV2"(w1242) -> ()
            n489 = local write "eV4"(w1242) -> ()
          }
          frame #1 {
            n490 = local read "MFC_1 User Set Value"() -> (w1257:dbl)
            n491 = local write "MFC_1\nSLPM Value"(w1257) -> ()
            n492 = Bundle(cluster=T4 {"Message"="", "Message Data"=variant} ("Message Cluster"), "Message"="MFC_1", "Message Data"=w1257) -> (w1260:T4)
            n493 = Enqueue Element(queue=w1262, element=w1260, error in (no error)=w1261) -> (queue out=w1259:refnum<queue>, error out=w1258:errorcluster)  [unwired: 1 in, 1 out]
          }
          frame #2 {
            n494 = for {
              N: 45 -> [w1271]
              i -> [w1270]
              n495 = Subtract(x=w1271, y=w1270) -> (x-y=w1269:i32)
              n496 = Decrement(x=w1269) -> (x-1=→"Low Cal\nFlush Time Remain (sec)":i32)
              n497 = Wait (ms)(milliseconds to wait=u32 1000) -> ()  [unwired: 1 out]
            }
          }
          frame #3 {
            w1275 = TRUE
            n498 = Bundle(cluster=T4 {"Message"="", "Message Data"=variant} ("Message Cluster"), "Message"="V1", "Message Data"=w1275) -> (w1278:T4)
            n499 = local write "eV1"(w1275) -> ()
            n500 = Enqueue Element(queue=w1277, element=w1278, error in (no error)=w1276) -> (queue out=w1274:refnum<queue>, error out=w1273:errorcluster)  [unwired: 1 in, 1 out]
          }
          frame #4 {
            n501 = for {
              N: 60 -> [w1287]
              i -> [w1286]
              n502 = Subtract(x=w1287, y=w1286) -> (x-y=w1285:i32)
              n503 = Decrement(x=w1285) -> (x-1=→"Low Cal\nCal Time Remain (sec)":i32)
              n504 = Wait (ms)(milliseconds to wait=u32 1000) -> ()  [unwired: 1 out]
            }
          }
          frame #5 {
            w1291 = FALSE
            n505 = Cluster To Array(cluster=T13 {"Message"="V2", "Message 3"="V4", "Message 4"="V1"}) -> (array=w1294:string[])
            n506 = for {
              tunnel: w1294 -> [w1301] mode=indexing
              tunnel: [w1300] -> w1290
              tunnel: [w1299] -> w1289
              tunnel: w1291 -> [w1298]
              tunnel: w1293 -> [w1297]
              tunnel: w1292 -> [w1296]
              n507 = Bundle(cluster=T4 {"Message"="", "Message Data"=variant} ("Message Cluster"), "Message"=w1301, "Message Data"=w1298) -> (w1303:T4)
              n508 = Enqueue Element(queue=w1297, element=w1303, error in (no error)=w1296) -> (queue out=w1300:refnum<queue>, error out=w1299:errorcluster)  [unwired: 1 in, 1 out]
            }
            n509 = local write "eV2"(w1291) -> ()
            n510 = local write "eV4"(w1291) -> ()
            n511 = local write "eV1"(w1291) -> ()
          }
          frame #6 {
            w1305 = 0.0 ("MFC_1\nSLPM Value")
            n512 = local write "MFC_1\nSLPM Value"(w1305) -> ()
            n513 = Bundle(cluster=T4 {"Message"="", "Message Data"=variant} ("Message Cluster"), "Message"="MFC_1", "Message Data"=w1305) -> (w1309:T4)
            n514 = Enqueue Element(queue=w1307, element=w1309, error in (no error)=w1306) -> (error out=w1304:errorcluster)  [unwired: 1 in, 2 out]
          }
          frame #7 {
            n515 = local write "Low Cal"(FALSE ("High Cal")) -> ()
          }
        }
      }
      event "Target Cal": Value Change {
        n516 = event-data() -> ()  [unwired: 1 in, 1 out]
        n517 = flat-sequence {
          tunnel: w1328 -> [w1336]
          tunnel: w1327 -> [w1335]
          tunnel: [w1334] -> w1326
          tunnel: [w1333] -> w1325
          tunnel: w1326 -> [w1342]
          tunnel: w1325 -> [w1341]
          tunnel: [w1339] -> w1323
          tunnel: [w1338] -> w1321
          tunnel: [w1347] -> w1324
          tunnel: w1323 -> [w1347]
          tunnel: [w1346] -> w1322
          tunnel: w1321 -> [w1346]
          tunnel: w1324 -> [w1357]
          tunnel: w1322 -> [w1356]
          tunnel: [w1354] -> w1319
          tunnel: [w1353] -> w1317
          tunnel: [w1363] -> w1320
          tunnel: w1319 -> [w1363]
          tunnel: [w1362] -> w1318
          tunnel: w1317 -> [w1362]
          tunnel: w1320 -> [w1372]
          tunnel: w1318 -> [w1371]
          tunnel: [w1369] -> w1316
          tunnel: [w1370] -> w1315
          tunnel: w1316 -> [w1387]
          tunnel: w1315 -> [w1386]
          tunnel: [w1384] -> w1313
          tunnel: [w1392] -> w1314
          tunnel: w1313 -> [w1392]
          frame #0 {
            w1332 = TRUE
            n518 = local write "eV4"(w1332) -> ()
            n519 = Bundle(cluster=T4 {"Message"="", "Message Data"=variant} ("Message Cluster"), "Message"="V4" ("Message 3"), "Message Data"=w1332) -> (w1331:T4)
            n520 = Enqueue Element(queue=w1336, element=w1331, error in (no error)=w1335) -> (queue out=w1334:refnum<queue>, error out=w1333:errorcluster)  [unwired: 1 in, 1 out]
          }
          frame #1 {
            n521 = local read "MFC_1 User Set Value"() -> (w1337:dbl)
            n522 = local write "MFC_1\nSLPM Value"(w1337) -> ()
            n523 = Bundle(cluster=T4 {"Message"="", "Message Data"=variant} ("Message Cluster"), "Message"="MFC_1", "Message Data"=w1337) -> (w1340:T4)
            n524 = Enqueue Element(queue=w1342, element=w1340, error in (no error)=w1341) -> (queue out=w1339:refnum<queue>, error out=w1338:errorcluster)  [unwired: 1 in, 1 out]
          }
          frame #2 {
            n525 = for {
              N: 45 -> [w1351]
              i -> [w1350]
              n526 = Subtract(x=w1351, y=w1350) -> (x-y=w1349:i32)
              n527 = Decrement(x=w1349) -> (x-1=→"Target Cal\nFlush Time Remain (sec)":i32)
              n528 = Wait (ms)(milliseconds to wait=u32 1000) -> ()  [unwired: 1 out]
            }
          }
          frame #3 {
            w1355 = TRUE
            n529 = Bundle(cluster=T4 {"Message"="", "Message Data"=variant} ("Message Cluster"), "Message"="V1", "Message Data"=w1355) -> (w1358:T4)
            n530 = local write "eV1"(w1355) -> ()
            n531 = Enqueue Element(queue=w1357, element=w1358, error in (no error)=w1356) -> (queue out=w1354:refnum<queue>, error out=w1353:errorcluster)  [unwired: 1 in, 1 out]
          }
          frame #4 {